vi "IMAQdx_AbsImage_Flea3_v4.4.vi"() -> ()   [LabVIEW 2012] (continued)
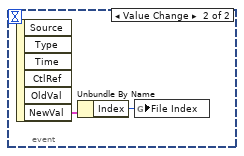
[diagram p3: hidden frame]
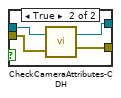
[diagram p5: hidden frame]
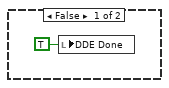
[diagram p6: hidden frame]
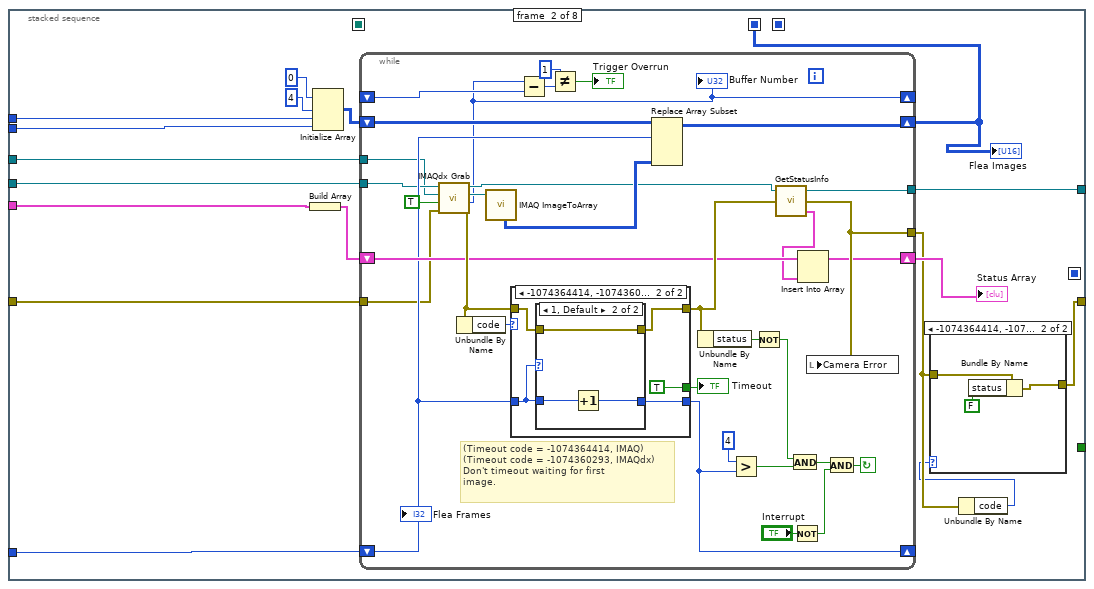
[diagram p7: hidden frame]
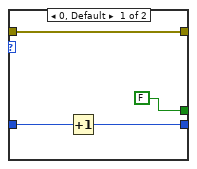
[diagram p9: hidden frame]
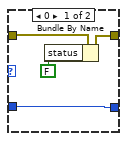
[diagram p10: hidden frame]
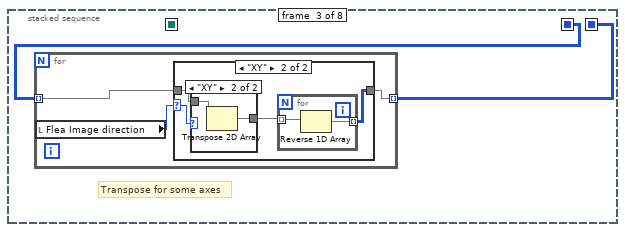
[diagram p11: hidden frame]
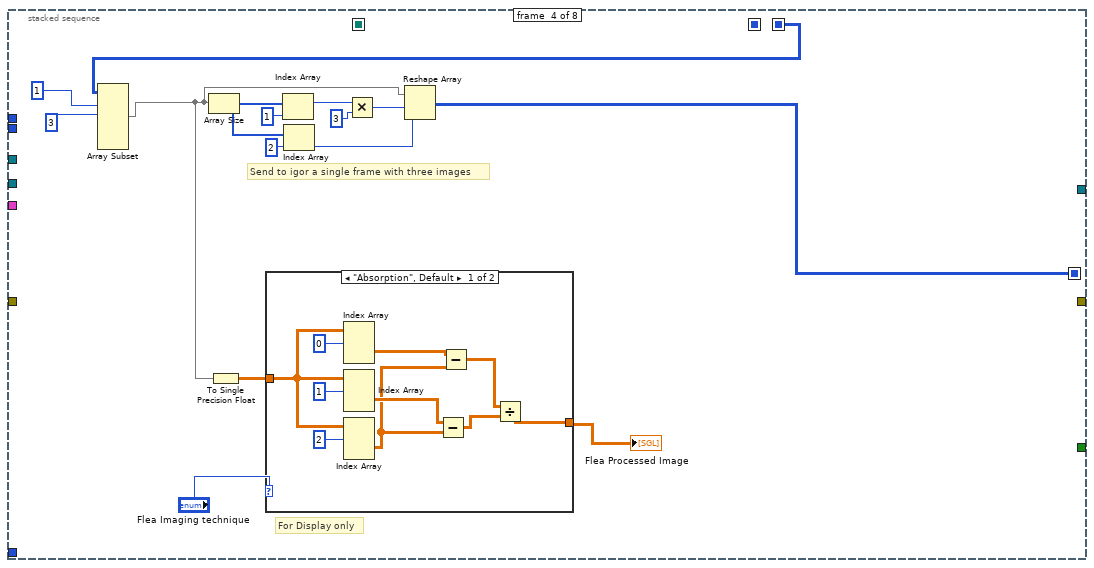
[diagram p14: hidden frame]
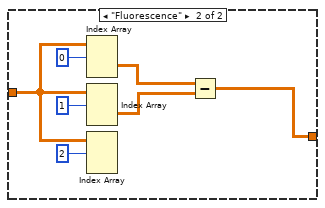
[diagram p15: hidden frame]
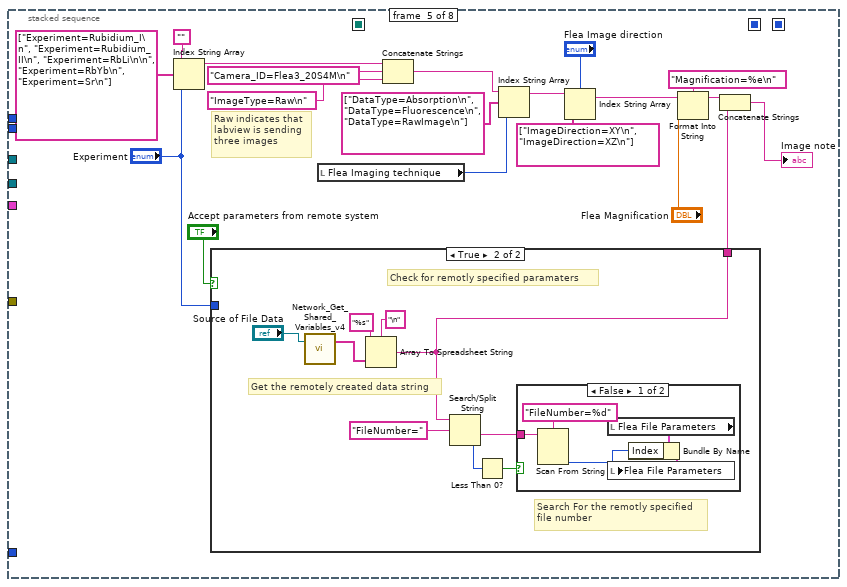
[diagram p16: hidden frame]
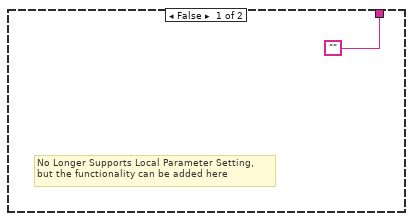
[diagram p17: hidden frame]
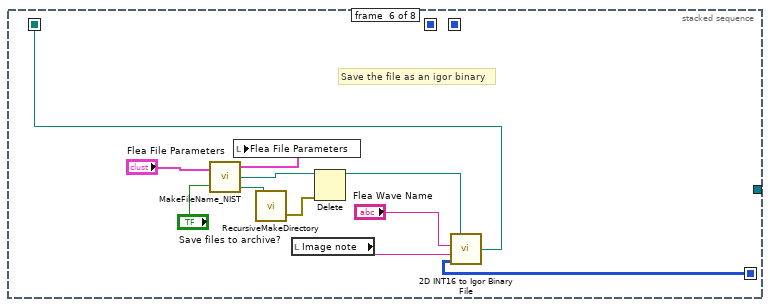
[diagram p19: hidden frame]
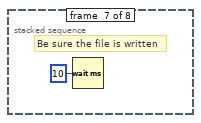
[diagram p20: hidden frame]
    tunnel: [w14] -> w6
    tunnel: ["SPE Load Error In"] -> w5
    tunnel: ["PIXIS Acquire"] -> w3
    tunnel: ["Flea Acquire"] -> w1
    tunnel: w7 -> [w28]
    tunnel: w8 -> [w26]
    tunnel: w6 -> [w27]
    tunnel: w5 -> [w25]
    tunnel: [w24] -> w4
    tunnel: w3 -> [w23]
    tunnel: [w22] -> w2
    tunnel: w1 -> [w21]
    tunnel: w4 -> [w451]
    tunnel: w2 -> [w450]
    frame #0 {
      w13 = T7 7 items=["Grayscale (U8)", "Grayscale (I16)", "Grayscale (SGL)", "Complex (CSG)", "RGB (U32)", "HSL (U32)", "RGB (U64)", "Grayscale (U16)"] ("Image Type")
      n2 = local read "Flea File Parameters"() -> (w17:T1)
      n3 = global write "FileInfo_Global.vi" "Lock File Number"(FALSE) -> ()
      n4 = Unbundle By Name(w17) -> ("Index"=w18:u32)
      n5 = global write "FileInfo_Global.vi" "File Index"(w18) -> ()
      n6 = call "IMAQ Create"("Image Name"="Camera Name", "Image Type"=w13) -> ("New Image"=w16:T8, "error out"=w14:errorcluster)  [unwired: 2 in, 1 out]
      n7 = local write "stop"(FALSE ("stop")) -> ()
      "Status" <- "Initializing..."
    }
    frame #1 {
      n8 = case shown="True" w21 {
        tunnel: w28 -> [_ w43]
        tunnel: w27 -> [w29 w42]
        tunnel: w26 -> [_ w40]
        tunnel: [w29 w32] -> w22
        frame False {
        }
        frame True {
          w50 = FALSE  # Debug?
          n9 = call "Setup For Triggered Images v4.2.vi"("error in"=w42, "Timeout (ms)"="Timeout (ms)", "Gain"="Gain", "Shutter speed"="Shutter speed", "Camera Name"=w43) -> ("Error out"=w51:errorcluster, "Session Out"=w52:T2, "Height"=w39:u32, "Width"=w38:u32)
          n10 = case shown="False" w50 {
            tunnel: [w58 w63] -> w49
            tunnel: [w59 w62] -> w46
            tunnel: w52 -> [w58 w61]
            tunnel: w51 -> [w59 w60]
            frame False {
            }
            frame True {
              n11 = call "CheckCameraAttributes-CDH.vi"("error in"=w60, "Camera Name"=w61) -> ("error out"=w62:errorcluster, "Session Out"=w63:T2)
            }
          }
          n12 = call "GetStatusInfo.vi"("error in"=w46, "Camera In"=w49) -> ("Status Info"=w37:T9, "error out"=w47:errorcluster, "Camera Out"=w48:T2)  [unwired: 1 in]
          n13 = call <vilib>:"IMAQdx Configure Acquisition.vi"("error in"=w47, "Number of Buffers"=u32 5, "Continuous?"=IMAQdx_Acquisition_Mode."Continuous", "Session In"=w48) -> ("error out"=w44:errorcluster, "Session Out"=w45:T2)  [unwired: 6 in]
          n14 = call <vilib>:"IMAQdx Start Acquisition.vi"("error in"=w44, "Session In"=w45) -> ("error out"=w35:errorcluster, "Session Out"=w41:T2)  [unwired: 8 out]
          n15 = while {
            tunnel: w41 -> [w73]
            tunnel: w40 -> [w72]
            tunnel: w39 -> [w71]
            tunnel: w38 -> [w70]
            tunnel: w37 -> [w69]
            tunnel: [w68] -> w31
            shift-right: [0] -> _
            shift-left: 0 -> [w67]
            shift-right: [w64] -> w34
            shift-left: w35 -> [w65]
            i -> [w75]
            stop <- w74 stop-if-true
            n16 = stacked-sequence {
              seq-local: [_ _ _ w178 _ _ _ _] -> [_ _ _ _ _ w236 _ _]
              seq-local: [_ _ _ _ _ w232 _ _] -> [_ _ _ _ _ _ _ w246]
              seq-local: [_ w81 _ _ _ _ _ _] -> [_ _ w152 _ _ _ _ _]
              seq-local: [_ _ w151 _ _ _ _ _] -> [_ _ _ w169 _ _ _ _]
              tunnel: [_ _ _ _ _ _ _ "stop"] -> w74
              tunnel: w73 -> [_ w93 _ _ _ _ _ _]
              tunnel: w72 -> [_ w92 _ _ _ _ _ _]
              tunnel: w71 -> [_ w91 _ _ _ _ _ _]
              tunnel: w70 -> [_ w90 _ _ _ _ _ _]
              tunnel: w69 -> [_ w88 _ _ _ _ _ _]
              tunnel: [_ w87 _ _ _ _ _ _] -> w68
              tunnel: [_ w84 _ _ _ _ _ _] -> w64
              tunnel: w67 -> [_ w86 _ _ _ _ _ _]
              tunnel: w65 -> [_ w85 _ _ _ _ _ _]
              frame #0 {
                n17 = local read "Send Flea data to Igor?"() -> (w76:bool)
                n18 = local write "Flea Frames"(0) -> ()
                n19 = local write "Status"("Running...") -> ()
                n20 = case shown="True" w76 {
                  frame False {
                    n21 = local write "DDE Done"(TRUE ("DDE Done")) -> ()
                  }
                  frame True {
                    "DDE Done" <- FALSE
                  }
                }
              }
              frame #1 {
                n22 = Build Array(w88) -> (w89:T4)
                n23 = Initialize Array(u16 0, 4, w91, w90) -> (w95:u16[][][])
                n24 = while {
                  shift-right: [w105] -> _
                  shift-left: _ -> [w129]
                  tunnel: [w113] -> w87
                  tunnel: [w110] -> w83
                  shift-right: [w120] -> _
                  shift-left: w86 -> [w107]
                  shift-right: [w125] -> w81
                  shift-left: w95 -> [w126]
                  shift-right: [w108] -> w94
                  shift-left: w89 -> [w109]
                  tunnel: w93 -> [w104]
                  tunnel: w92 -> [w103]
                  tunnel: w85 -> [w102]
                  stop <- w116 continue-if-true
                  # "(Timeout code = -1074364414, IMAQ)\n(Timeout code = -1074360293, IMAQdx)\nDon't timeout waiting for first\nimage."
                  n25 = call <vilib>:"IMAQdx Grab.vi"("error in"=w102, "Wait for Next Buffer? (Yes)"=TRUE, "Image In"=w103, "Session In"=w104) -> ("error out"=w124:errorcluster, "Buffer Number Out"=w105:u32, "Image Out"=w119:T8, "Session Out"=w112:T2)  [unwired: 4 out]
                  "Buffer Number" <- w105
                  n26 = Unbundle By Name(w124) -> ("code"=w133:i32)
                  n27 = call "IMAQ ImageToArray"("Image"=w119) -> ("Image Pixels (U16)"=w118:u16[][])  [unwired: 2 in, 5 out]
                  n28 = case shown="-1074364414, -1074360293" w133 {
                    tunnel: w124 -> [w138 w142]
                    tunnel: [w138 w141] -> w111
                    tunnel: [FALSE TRUE] -> w134
                    tunnel: w107 -> [w136 w140]
                    tunnel: [w135 w139] -> w120
                    frame 0, Default {
                      n29 = Increment(x=w136) -> (x+1=w135:i32)
                    }
                    frame -1074364414, -1074360293 {
                      n30 = case shown="1, Default" w140 {
                        tunnel: [w144 w150] -> w141
                        tunnel: w142 -> [w146 w150]
                        tunnel: w140 -> [w145 w149]
                        tunnel: [w145 w148] -> w139
                        frame 0 {
                          n31 = Bundle By Name(cluster=w146, "status"=FALSE) -> (w144:errorcluster)
                        }
                        frame 1, Default {
                          n32 = Increment(x=w149) -> (x+1=w148:i32)
                        }
                      }
                    }
                  }
                  "Timeout" <- w134
                  n33 = Subtract(x=w105, y=w129) -> (x-y=w130:u32)
                  n34 = Not Equal?(x=u32 1, y=w130) -> (x != y?=→"Trigger Overrun":bool)
                  n35 = Replace Array Subset(array=w126, new element=w118, index (dim 0)=w107) -> (w125:u16[][][])  [unwired: 2 in]
                  n36 = Unbundle By Name(w111) -> ("status"=w128:bool)
                  n37 = Greater?(x=4, y=w120) -> (0:w121:bool)
                  n38 = Not(x=w128) -> (.not. x?=w127:bool)
                  n39 = call "GetStatusInfo.vi"("error in"=w111, "Camera In"=w112) -> ("Status Info"=w106:T9, "error out"=w110:errorcluster, "Camera Out"=w113:T2)  [unwired: 1 in]
                  n40 = And(x=w127, y=w121) -> (x .and. y?=w117:bool)
                  n41 = Not(x="Interrupt") -> (.not. x?=w114:bool)
                  n42 = Insert Into Array(array=w109, new element=w106) -> (w108:T4)  [unwired: 1 in]
                  n43 = local write "Camera Error"(w110) -> ()
                  n44 = And(x=w117, y=w114) -> (x .and. y?=w116:bool)
                  "Flea Frames" <- w107
                }
                "Flea Images" <- w81
                "Status Array" <- w94
                n45 = Unbundle By Name(w83) -> ("code"=w82:i32)
                n46 = case shown="-1074364414, -1074360293" w82 {
                  tunnel: [w98 w100] -> w84
                  tunnel: w83 -> [w98 w99]
                  frame 0, Default {
                  }
                  frame -1074364414, -1074360293 {
                    n47 = Bundle By Name(cluster=w99, "status"=FALSE) -> (w100:errorcluster)
                  }
                }
              }
              frame #2 {
                # "Transpose for some axes"
                n48 = for {
                  tunnel: w152 -> [w154] mode=indexing
                  tunnel: [w153] -> w151 mode=indexing
                  n49 = local read "Flea Image direction"() -> (w155:enum16{"XY", "XZ"})
                  n50 = case shown="\"XY\"" w155 {
                    selector: w155 -> [_ w157]
                    tunnel: w154 -> [w156 w159]
                    tunnel: [w156 w160] -> w153
                    frame Default {
                    }
                    frame "XY" {
                      n51 = case shown="\"XY\"" w157 {
                        tunnel: w159 -> [w161 w163]
                        tunnel: [w161 w162] -> w158
                        frame Default {
                        }
                        frame "XY" {
                          n52 = Transpose 2D Array(2D array=w163) -> (transposed array=w162:u16[][])
                        }
                      }
                      n53 = for {
                        tunnel: w158 -> [w165] mode=indexing
                        tunnel: [w164] -> w160 mode=indexing
                        n54 = Reverse 1D Array(array=w165) -> (reversed array=w164:u16[])
                      }
                    }
                  }
                }
              }
              frame #3 {
                # "Send to igor a single frame with three images"
                # "For Display only"
                n55 = Array Subset(array=w169, index (dim 0)=1 ("index"), length (dim 0)=3 ("length")) -> (w166:u16[][][])  [unwired: 4 in]
                n56 = Array Size(array=w166) -> (size(s)=w174:i32[])
                n57 = To Single Precision Float(number=w166) -> (single precision float=w175:sgl[][][])
                n58 = case shown="\"Absorption\", Default" "Flea Imaging technique" {
                  tunnel: [w187 w193] -> w179
                  tunnel: w175 -> [w186 w194]
                  frame "Absorption", Default {
                    n59 = Index Array(array=w186, index (dim 0)=0 ("Number of buffers")) -> (element=w185:sgl[][])  [unwired: 2 in]
                    n60 = Index Array(array=w186, index (dim 0)=1 ("Number of buffers")) -> (element=w184:sgl[][])  [unwired: 2 in]
                    n61 = Index Array(array=w186, index (dim 0)=2 ("Number of buffers")) -> (element=w183:sgl[][])  [unwired: 2 in]
                    n62 = Subtract(x=w184, y=w183) -> (x-y=w182:sgl[][])
                    n63 = Subtract(x=w185, y=w183) -> (x-y=w181:sgl[][])
                    n64 = Divide(x=w181, y=w182) -> (x/y=w187:sgl[][])
                  }
                  frame "Fluorescence" {
                    n65 = Index Array(array=w194, index (dim 0)=0 ("Number of buffers")) -> (element=w192:sgl[][])  [unwired: 2 in]
                    n66 = Index Array(array=w194, index (dim 0)=1 ("Number of buffers")) -> (element=w191:sgl[][])  [unwired: 2 in]
                    n67 = Index Array(array=w194, index (dim 0)=2 ("Number of buffers")) -> ()  [unwired: 2 in, 1 out]
                    n68 = Subtract(x=w192, y=w191) -> (x-y=w193:sgl[][])
                  }
                }
                "Flea Processed Image" <- w179
                n69 = Index Array(array=w174, index=1 ("Number of buffers")) -> (element=w171:i32)
                n70 = Index Array(array=w174, index=2 ("Number of buffers")) -> (element=w170:i32)
                n71 = Multiply(x=w171, y=3 ("Number of buffers")) -> (x*y=w176:i32)
                n72 = Reshape Array(w166, w176, w170) -> (w178:u16[][])
              }
              frame #4 {
                # "Raw indicates that\nlabview is sending\nthree images"
                n73 = Index String Array(1:"Experiment", 2:string[] ["Experiment=Rubidium_I\n", "Experiment=Rubidium_II\n", "Experiment=RbLi\n\n", "Experiment=RbYb\n", "Experiment=Sr\n"], 3:"") -> (0:w202:string)
                n74 = case shown="True" "Accept parameters from remote system" {
                  tunnel: ["" w219] -> w208
                  tunnel: "Experiment" -> [_ _]
                  frame False {
                    # "No Longer Supports Local Parameter Setting,\nbut the functionality can be added here"
                  }
                  frame True {
                    # "Check for remotly specified paramaters"
                    # "Get the remotely created data string"
                    # "Search For the remotly specified\nfile number"
                    n75 = call "Network_Get_Shared_Variables_v4.vi"("Source of Data"="Source of File Data") -> ("Igor Instruction String"=w226:string[])  [unwired: 1 in, 1 out]
                    n76 = Array To Spreadsheet String(delimiter (Tab)="\n", array=w226, 3:"%s") -> (spreadsheet string=w219:string)
                    n77 = Search/Split String(string=w219, search string/char (-)="FileNumber=") -> (match + rest of string=w222:string, offset of match=w221:i32)  [unwired: 2 out]
                    n78 = Less Than 0?(x=w221) -> (x < 0?=w220:bool)
                    n79 = case shown="False" w220 {
                      tunnel: w222 -> [w231 _]
                      frame False {
                        n80 = Scan From String(format string="FileNumber=%d", input string=w231) -> (output 1=w227:i32)  [unwired: 2 in, 4 out]
                        n81 = local read "Flea File Parameters"() -> (w229:T1)
                        n82 = Bundle By Name(cluster=w229, "Index"=w227) -> (w228:T1)
                        n83 = local write "Flea File Parameters"(w228) -> ()
                      }
                      frame True {
                      }
                    }
                  }
                }
                n84 = local read "Flea Imaging technique"() -> (w213:enum16{"Absorption", "Fluorescence", "RawImage"})
                n85 = Concatenate Strings(w202, "Camera_ID=Flea3_20S4M\n", "ImageType=Raw\n") -> (w203:string)
                n86 = Index String Array(1:w213, 2:string[] ["DataType=Absorption\n", "DataType=Fluorescence\n", "DataType=RawImage\n"], 3:w203) -> (0:w214:string)
                n87 = Index String Array(1:"Flea Image direction", 2:string[] ["ImageDirection=XY\n", "ImageDirection=XZ\n"], 3:w214) -> (0:w216:string)
                n88 = Format Into String(format string="Magnification=%e\n", initial string=w216, "Flea Magnification") -> (resulting string=w210:string)  [unwired: 1 in, 1 out]
                n89 = Concatenate Strings(w210, w208) -> (→"Image note":string)
              }
              frame #5 {
                # "Save the file as an igor binary"
                n90 = call "MakeFileName_NIST.vi"("File Parameters"="Flea File Parameters", "Save permanent file?"="Save files to archive?") -> ("New file parameters."=w238:T1, "Path to File"=w240:path, "path"=w239:path)
                n91 = local write "Flea File Parameters"(w238) -> ()
                n92 = call "RecursiveMakeDirectory.vi"("Directory to create"=w239) -> ("error out"=w242:errorcluster)  [unwired: 1 in, 1 out]
                n93 = local read "Image note"() -> (w235:string)
                n94 = Delete(path (use dialog)=w240, error in=w242) -> (deleted path=w233:path)  [unwired: 5 out]
                n95 = call "2D INT16 to Igor Binary File.vi"("Wave Data (I16)"=w236, "Wave Note (\"\")"=w235, "WaveName"="Flea Wave Name", "Path (default: dialog)"=w233) -> ("Path chosen"=w232:path)
              }
              frame #6 {
                # "Be sure the file is written"
                n96 = Wait (ms)(milliseconds to wait=u32 10) -> ()  [unwired: 1 out]
              }
              frame #7 {
                n97 = case shown="True" "Send Flea data to Igor?" {
                  tunnel: w246 -> [_ w258]
                  tunnel: ["" w250] -> w245
                  frame False {
                  }
                  frame True {
                    n98 = local read "Send PIXIS data to Igor?"() -> (w253:bool)
                    n99 = flat-sequence {
                      tunnel: w249 -> [w259]
                      frame #0 {
                        # "Tell Igor what file to open"
                        n100 = call <vilib>:"DDE Open Conversation.vi"("topic"="Igor", "service"="Igor") -> ("error out"=w263:errorcluster, "conversation refnum"=w265:u32)  [unwired: 1 in, 5 out]
                        n101 = call <vilib>:"DDE Execute.vi"("error in (no error)"=w263, "command"=w259, "conversation refnum in"=w265) -> ("error out"=w264:errorcluster, "conversation refnum out"=w266:u32)  [unwired: 5 out]
                        n102 = call <vilib>:"DDE Close Conversation.vi"("error in (no error)"=w264, "conversation refnum"=w266) -> ("error out"=→"DDE Error":errorcluster)  [unwired: 7 out]
                      }
                      frame #1 {
                        n103 = local write "DDE Done"(TRUE ("Waiting for Flea File")) -> ()
                      }
                      frame #2 {
                        n104 = Wait (ms)(milliseconds to wait=u32 50) -> ()  [unwired: 1 out]
                      }
                    }
                    n105 = Path To String(path=w258) -> (string=w257:string)
                    n106 = Search and Replace String(replace all?=TRUE, input string=w257, search string="\\", replace string="\\\\") -> (result string=w252:string)  [unwired: 1 in, 6 out]
                    n107 = case shown="True" w253 {
                      tunnel: w252 -> [w271 w275]
                      tunnel: "Flea Data Series Name" -> [w272 w278]
                      tunnel: [w269 w276] -> w250
                      tunnel: [w269 w276] -> w249
                      frame False {
                        n108 = Format Into String(format string="AutoRunV3(\"%s\",\"%s\") ", w272, w271) -> (resulting string=w269:string)  [unwired: 2 in, 1 out]
                      }
                      frame True {
                        n109 = local read "PIXIS Data Series Name"() -> (w274:string)
                        n110 = stacked-sequence {
                          tunnel: [_ w281] -> w273
                          frame #0 {
                            n111 = while {
                              stop <- w280 continue-if-true
                              n112 = local read "Waiting for PIXIS file"() -> (w280:bool)
                              n113 = Wait (ms)(milliseconds to wait=u32 5) -> ()  [unwired: 1 out]
                            }
                          }
                          frame #1 {
                            n114 = local read "PIXIS Path"() -> (w286:path)
                            n115 = Path To String(path=w286) -> (string=w282:string)
                            n116 = Search and Replace String(replace all?=TRUE, input string=w282, search string="\\", replace string="\\\\") -> (result string=w281:string)  [unwired: 1 in, 6 out]
                          }
                        }
                        n117 = Format Into String(format string="AutoRunV4(\"%s\",\"%s\",\"%s\",\"%s\") ", w278, w275, w274, w273) -> (resulting string=w276:string)  [unwired: 2 in, 1 out]
                      }
                    }
                  }
                }
                "Command to Igor" <- w245
                "Flea Path" <- w246
              }
            }
            "Flea Loop" <- w75
          }
          n118 = call <vilib>:"IMAQdx Unconfigure Acquisition.vi"("error in"=w34, "Session In"=w31) -> ("error out"=w33:errorcluster, "Session Out"=w30:T2)  [unwired: 8 in]
          n119 = call <vilib>:"IMAQdx Close Camera.vi"("error in"=w33, "Session In"=w30) -> ("error out"=w32:errorcluster)  [unwired: 9 out]
        }
      }
      n120 = case shown="True" w23 {
        tunnel: w25 -> [w287 w289]
        tunnel: [w287 w288] -> w24
        frame False {
        }
        frame True {
          n121 = while {
            tunnel: [w291] -> w288
            tunnel: w289 -> [w293]
            i -> [w294]
            stop <- w292 stop-if-true
            n122 = stacked-sequence {
              seq-local: [_ _ w343 _ _ _ _] -> [_ _ _ _ w401 _ _]
              seq-local: [_ _ _ _ w397 _ _] -> [_ _ _ _ _ _ w417]
              seq-local: [_ w301 _ _ _ _ _] -> [_ _ w331 _ _ _ _]
              seq-local: [_ w299 _ _ _ _ _] -> [_ _ _ _ _ _ w411]
              seq-local: [_ w298 _ _ _ _ _] -> [_ _ _ _ _ _ w410]
              tunnel: w293 -> [_ w300 _ _ _ _ _]
              tunnel: [_ _ _ _ _ _ w412] -> w292
              tunnel: [_ _ _ _ _ _ w409] -> w291
              tunnel: [_ _ _ _ _ _ w408] -> w290
              frame #0 {
                n123 = local write "Status"("Running...") -> ()
                n124 = local write "PIXIS Frames"(i64 0) -> ()
                "Waiting for PIXIS file" <- TRUE
              }
              frame #1 {
                n125 = while {
                  tunnel: "SPE File Path" -> [w321]
                  shift-right: [w320] -> w311
                  shift-left: w300 -> [w317]
                  tunnel: [w318] -> w303
                  tunnel: "Source of Control Data" -> [w313]
                  stop <- w319 stop-if-true
                  n126 = local read "CycleDone"() -> (w316:bool)
                  n127 = DataSocket Read(8:w317, 10:w316, 11:w313) -> (0:w315:errorcluster, 2:w314:bool)  [unwired: 2 in, 5 out]
                  "CycleDone" <- w314
                  "DS Error" <- w315
                  n128 = case shown="True" w314 {
                    tunnel: w321 -> [w324 w329]
                    tunnel: [w323 w328] -> w320
                    tunnel: [FALSE ("file or folder exists?") w327] -> w319
                    tunnel: [w324 w326] -> w318
                    tunnel: w315 -> [w323 w325]
                    frame False {
                    }
                    frame True {
                      n129 = call <vilib>:"Check if File or Folder Exists.vi"("error in (no error)"=w325, "path"=w329) -> ("error out"=w328:errorcluster, "file or folder exists?"=w327:bool, "dup path"=w326:path)  [unwired: 7 in]
                    }
                  }
                }
                n130 = call "Load SPE v0.2.vi"("Error In"=w311, "File Path In"=w303) -> ("Error Out"=w298:errorcluster, "DataBlock Info"=w305:T5, "Output Stack"=w308:cluster{u16[][][]}[], "File Path Out"=w299:path, "Parse Errors"=→"XML Parse Errors":string)  [unwired: 5 in]
                "DataBlock Info" <- w305
                n131 = Unbundle By Name(w305) -> ("frame count"=→"PIXIS Frames":i64)
                n132 = Index Array(array=w308, index=0) -> (element=w306:cluster{u16[][][]})
                n133 = Array Size(array=w308) -> (size(s)=→"Data Array Size":i32)
                n134 = Unbundle(w306) -> (w301:u16[][][])
                "PIXIS Images" <- w301
              }
              frame #2 {
                # "Send to igor a single frame with three images"
                # "For Display only"
                n135 = Array Subset(array=w331, index (dim 0)=1 ("index"), length (dim 0)=3 ("length")) -> (w332:u16[][][])  [unwired: 4 in]
                n136 = Array Size(array=w332) -> (size(s)=w339:i32[])
                n137 = To Single Precision Float(number=w332) -> (single precision float=w340:sgl[][][])
                n138 = case shown="\"Absorption\", Default" "PIXIS Imaging technique" {
                  tunnel: [w350 w357] -> w330
                  tunnel: w340 -> [w351 w358]
                  frame "Absorption", Default {
                    n139 = Index Array(array=w351, index (dim 0)=0 ("Number of buffers")) -> (element=w347:sgl[][])  [unwired: 2 in]
                    n140 = Index Array(array=w351, index (dim 0)=1 ("Number of buffers")) -> (element=w345:sgl[][])  [unwired: 2 in]
                    n141 = Index Array(array=w351, index (dim 0)=2 ("Number of buffers")) -> (element=w346:sgl[][])  [unwired: 2 in]
                    n142 = Subtract(x=w345, y=w346) -> (x-y=w349:sgl[][])
                    n143 = Subtract(x=w347, y=w346) -> (x-y=w348:sgl[][])
                    n144 = Divide(x=w348, y=w349) -> (x/y=w350:sgl[][])
                  }
                  frame "Fluorescence" {
                    n145 = Index Array(array=w358, index (dim 0)=0 ("Number of buffers")) -> (element=w356:sgl[][])  [unwired: 2 in]
                    n146 = Index Array(array=w358, index (dim 0)=1 ("Number of buffers")) -> (element=w355:sgl[][])  [unwired: 2 in]
                    n147 = Index Array(array=w358, index (dim 0)=2 ("Number of buffers")) -> ()  [unwired: 2 in, 1 out]
                    n148 = Subtract(x=w356, y=w355) -> (x-y=w357:sgl[][])
                  }
                }
                "PIXIS Processed Image" <- w330
                n149 = Index Array(array=w339, index=1 ("Number of buffers")) -> (element=w336:i32)
                n150 = Index Array(array=w339, index=2 ("Number of buffers")) -> (element=w335:i32)
                n151 = Multiply(x=w336, y=3 ("Number of buffers")) -> (x*y=w341:i32)
                n152 = Reshape Array(w332, w341, w335) -> (w343:u16[][])
              }
              frame #3 {
                # "Raw indicates that\nlabview is sending\nthree images"
                n153 = local read "Accept parameters from remote system"() -> (w362:bool)
                n154 = local read "Experiment"() -> (w363:T3)
                n155 = Index String Array(1:w363, 2:string[] ["Experiment=Rubidium_I\n", "Experiment=Rubidium_II\n", "Experiment=RbLi\n\n", "Experiment=RbYb\n", "Experiment=Sr\n"], 3:"") -> (0:w367:string)
                n156 = case shown="True" w362 {
                  tunnel: ["" w383] -> w372
                  tunnel: w363 -> [_ _]
                  frame False {
                    # "No Longer Supports Local Parameter Setting,\nbut the functionality can be added here"
                  }
                  frame True {
                    # "Check for remotely specified paramaters"
                    # "Get the remotely created data string"
                    # "Search For the remotly specified\nfile number"
                    n157 = local read "Source of File Data"() -> (w382:refnum<k21>)
                    n158 = call "Network_Get_Shared_Variables_v4.vi"("Source of Data"=w382) -> ("Igor Instruction String"=w390:string[])  [unwired: 1 in, 1 out]
                    n159 = Array To Spreadsheet String(delimiter (Tab)="\n", array=w390, 3:"%s") -> (spreadsheet string=w383:string)
                    n160 = Search/Split String(string=w383, search string/char (-)="FileNumber=") -> (match + rest of string=w386:string, offset of match=w385:i32)  [unwired: 2 out]
                    n161 = Less Than 0?(x=w385) -> (x < 0?=w384:bool)
                    n162 = case shown="False" w384 {
                      tunnel: w386 -> [w395 _]
                      frame False {
                        n163 = Scan From String(format string="FileNumber=%d", input string=w395) -> (output 1=w391:i32)  [unwired: 2 in, 4 out]
                        n164 = local read "PIXIS File Parameters"() -> (w393:T1)
                        n165 = Bundle By Name(cluster=w393, "Index"=w391) -> (w392:T1)
                        n166 = local write "PIXIS File Parameters"(w392) -> ()
                      }
                      frame True {
                      }
                    }
                  }
                }
                n167 = local read "PIXIS Imaging technique"() -> (w377:enum16{"Absorption", "Fluorescence", "RawImage"})
                n168 = Concatenate Strings(w367, "Camera_ID=PIXIS\n", "ImageType=Raw\n") -> (w368:string)
                n169 = Index String Array(1:w377, 2:string[] ["DataType=Absorption\n", "DataType=Fluorescence\n", "DataType=RawImage\n"], 3:w368) -> (0:w378:string)
                n170 = Index String Array(1:"PIXIS Image direction", 2:string[] ["ImageDirection=XY\n", "ImageDirection=XZ\n"], 3:w378) -> (0:w380:string)
                n171 = Format Into String(format string="Magnification=%e\n", initial string=w380, "PIXIS Magnification") -> (resulting string=w374:string)  [unwired: 1 in, 1 out]
                n172 = Concatenate Strings(w374, w372) -> (→"PIXIS Image Note":string)
              }
              frame #4 {
                # "Save the file as an igor binary"
                n173 = local read "Save files to archive?"() -> (w396:bool)
                n174 = call "MakeFileName_NIST.vi"("File Parameters"="PIXIS File Parameters", "Save permanent file?"=w396) -> ("New file parameters."=w403:T1, "Path to File"=w405:path, "path"=w404:path)
                n175 = local write "PIXIS File Parameters"(w403) -> ()
                n176 = call "RecursiveMakeDirectory.vi"("Directory to create"=w404) -> ("error out"=w406:errorcluster)  [unwired: 1 in, 1 out]
                n177 = local read "PIXIS Image Note"() -> (w400:string)
                n178 = Delete(path (use dialog)=w405, error in=w406) -> (deleted path=w398:path)  [unwired: 5 out]
                n179 = call "2D INT16 to Igor Binary File.vi"("Wave Data (I16)"=w401, "Wave Note (\"\")"=w400, "WaveName"="PIXIS Wave Name", "Path (default: dialog)"=w398) -> ("Path chosen"=w397:path)
              }
              frame #5 {
                # "Be sure the file is written"
                n180 = Wait (ms)(milliseconds to wait=u32 10) -> ()  [unwired: 1 out]
              }
              frame #6 {
                n181 = local read "Send Flea data to Igor?"() -> (w413:bool)
                n182 = Not(x=w413) -> (.not. x?=w416:bool)
                n183 = And(x="Send PIXIS data to Igor?", y=w416) -> (x .and. y?=w414:bool)
                n184 = case shown="False" w414 {
                  tunnel: w417 -> [_ w441]
                  tunnel: w411 -> [w420 w430]
                  tunnel: w410 -> [w419 w431]
                  tunnel: [w421 w432] -> w409
                  tunnel: [w418 w429] -> w408
                  frame False {
                    n185 = stacked-sequence {
                      tunnel: [w425 _] -> w421
                      tunnel: w420 -> [w424 _]
                      tunnel: w419 -> [w423 _]
                      tunnel: [w422 _] -> w418
                      frame #0 {
                        n186 = local write "Waiting for PIXIS file"(FALSE ("Waiting for PIXIS file")) -> ()
                        n187 = Delete(path (use dialog)=w424, error in=w423) -> (deleted path=w422:path, error out=w425:errorcluster)  [unwired: 3 in, 1 out]
                      }
                      frame #1 {
                        n188 = while {
                          stop <- w427 stop-if-true
                          n189 = local read "DDE Done"() -> (w427:bool)
                          n190 = Wait (ms)(milliseconds to wait=u32 5) -> ()  [unwired: 1 out]
                        }
                      }
                    }
                  }
                  frame True {
                    # "Tell Igor what file to open"
                    n191 = Path To String(path=w441) -> (string=w440:string)
                    n192 = call <vilib>:"DDE Open Conversation.vi"("topic"="Igor", "service"="Igor") -> ("error out"=w445:errorcluster, "conversation refnum"=w443:u32)  [unwired: 1 in, 5 out]
                    n193 = Search and Replace String(replace all?=TRUE, input string=w440, search string="\\", replace string="\\\\") -> (result string=w436:string)  [unwired: 1 in, 6 out]
                    n194 = Format Into String(format string="AutoRunV3(\"%s\",\"%s\") ", "PIXIS Data Series Name", w436) -> (resulting string=w434:string)  [unwired: 2 in, 1 out]
                    n195 = call <vilib>:"DDE Execute.vi"("error in (no error)"=w445, "command"=w434, "conversation refnum in"=w443) -> ("error out"=w444:errorcluster, "conversation refnum out"=w442:u32)  [unwired: 5 out]
                    n196 = local write "Command to Igor"(w434) -> ()
                    n197 = call <vilib>:"DDE Close Conversation.vi"("error in (no error)"=w444, "conversation refnum"=w442) -> ("error out"=w433:errorcluster)  [unwired: 7 out]
                    n198 = local write "DDE Error"(w433) -> ()
                    n199 = Delete(path (use dialog)=w430, error in=w431) -> (deleted path=w429:path, error out=w432:errorcluster)  [unwired: 3 in, 1 out]
                  }
                }
                n200 = local read "stop"() -> (w412:bool)
                "PIXIS Path" <- w417
              }
            }
            "SPE delete path" <- w290
            "PIXIS Loop" <- w294
          }
        }
      }
    }
    frame #2 {
      n201 = local write "stop"(FALSE ("stop")) -> ()
      n202 = local write "Status"("Done.") -> ()
      "Camera Error" <- w450
      "SPE Load Error Out" <- w451
    }
    frame #3 {
      n203 = Stop() -> ()  [unwired: 1 out]
    }
  }
  n204 = while {
    stop <- TRUE continue-if-true
    n205 = event shown="[0] \"Flea Raw image to view\", \"Flea Images\", \"Update Graphics\", \"PIXIS Raw image to view\", \"PIXIS Images\": Value Change;  Timeout" {
      selector: _ -> [_ _]
      dyn-events: _ -> [_ _]
      timeout: 1000 -> [_ _]
      event "Flea Raw image to view", "Flea Images", "Update Graphics", "PIXIS Raw image to view", "PIXIS Images": Value Change; Timeout {
        n206 = event-data() -> ()  [unwired: 4 out]
        n207 = case shown="True" "Update Graphics" {
          frame False {
          }
          frame True {
            n208 = local read "Flea Images"() -> (w461:u16[][][])
            n209 = local read "PIXIS Images"() -> (w456:u16[][][])
            n210 = Index Array(array=w461, index (dim 0)="Flea Raw image to view") -> (element=→"Flea Raw Image":u16[][])  [unwired: 2 in]
            n211 = Index Array(array=w456, index (dim 0)="PIXIS Raw image to view") -> (element=→"PIXIS Raw Image":u16[][])  [unwired: 2 in]
          }
        }
      }
      event Value Change {
        n212 = event-data() -> ("NewVal"=w462:T1)  [unwired: 6 out]
        n213 = Unbundle By Name(w462) -> ("Index"=w463:u32)
        n214 = global write "FileInfo_Global.vi" "File Index"(w463) -> ()
      }
    }
  }
